vi "CRYO_MASTER_FULL_dev.vi"() -> ()   [LabVIEW 2017]
uses:
  LSI218Data.lvclass
  LSI336Data.lvclass
  USBData.lvclass
  6240AData.lvclass
  DMMsData.lvclass
  LMData.lvclass
  <vilib>/DAQmx/miscellaneous.llb/DAQmx Fill In Error Info.vi
  <vilib>/DAQmx/create/channels.llb/DAQmx Create Channel (DO-Digital Output).vi
  <vilib>/DAQmx/create/channels.llb/DAQmx Create Channel (AO-Voltage-Basic).vi
  <vilib>/express/express arith-compare/Formula/XNode/ExpressFormulaBlockNode.xnode
  <vilib>/Analysis/NI_AALBase.lvlib
  istr.lib/Agilent 33XXX Series/Agilent 33XXX Series.lvlib
panel:
  in  "Automatic \nScreenshots?":bool=TRUE
  in  "Frontpanel screenshots":bool
  in  "Screenshots interval":i64=3605
  in  "Record interval":i64=10
  out "Cycle #":u32
  in  "Measurement Interval (s)":dbl=1.0
  in  "Stop Button":bool
  in  "?":T1(tab)=enum."INST CONFIG"
  out "RUN Identifier":string="20201120_195613_RUNII"
  in  "Base Path (screenshots)":path=path "C:/LabVIEW/DATA/Google/TUCAN Experiments/KEK_cryotests_2019-2020/data/screenshots"
  out "error out (USB6210/6218 AOUT)":errorcluster
  in  "AOUT Labels":string[](array[string])=["PWR400H_I", "PMC183A_I"]
  in  "DOUT Labels":string[](array[string])=["D_V1_NO", "D_V2_NC", "D_CV1", "D_H1"]
  in  "AOUT assignment":tag[](array[tag])=["Dev1/ao0", "Dev1/ao1"]
  out "AO task out":refnum<k21>="20201120_102906_RUNII_AO"
  in  "Analog Out ON?":bool=TRUE
  in  "InstName (USB6218)":string="USB6218"
  in  "USB6218 Config":T2(array[cluster])=[{"Label"="F_1", "FileFormat"="%5.5f", "Active?"=TRUE, "Physical CH"="Dev1/ai0", " terminal\n type"=10083, "ConversionType"={"Type"=enum."SimpleProp", "ConversionParameters"=[0.0, 5.0, 0.0, 500.0]}, "VoltageLimits"=[0.0, 5.0]}, {"Label"="F_2", "FileFormat"="%5.5f", "Active?"=TRUE, "Physical CH"="Dev1/ai1", " terminal\n type"=10083, "ConversionType"={"Type"=enum."SimpleProp", "ConversionParameters"=[0.0, 5.0, 0.0, 200.0]}, "VoltageLimits"=[0.0, 5.0]}, {"Label"="F_3", "FileFormat"="%5.5f", "Active?"=TRUE, "Physical CH"="Dev1/ai2", " terminal\n type"=10083, "ConversionType"={"Type"=enum."SimpleProp", "ConversionParameters"=[0.0, 5.0, 0.0, 200.0]}, "VoltageLimits"=[0.0, 5.0]}, {"Label"="F_4", "FileFormat"="%5.5f", "Active?"=TRUE, "Physical CH"="Dev1/ai3", " terminal\n type"=10083, "ConversionType"={"Type"=enum."SimpleProp", "ConversionParameters"=[0.0, 5.0, 0.0, 500.0]}, "VoltageLimits"=[0.0, 5.0]}, {"Label"="F_5", "FileFormat"="%5.5f", "Active?"=TRUE, "Physical CH"="Dev1/ai4", " terminal\n type"=10083, "ConversionType"={"Type"=enum."SimpleProp", "ConversionParameters"=[0.0, 5.0, 0.0, 500.0]}, "VoltageLimits"=[0.0, 5.0]}, {"Label"="I_CV", "FileFormat"="%3.5f", "Active?"=TRUE, "Physical CH"="Dev1/ai5", " terminal\n type"=10083, "ConversionType"={"Type"=enum."Raw", "ConversionParameters"=[0.0, 0.0, 0.0, 0.0]}, "VoltageLimits"=[0.0, 10.0]}, {"Label"="CV1_answer", "FileFormat"="%3.5f", "Active?"=TRUE, "Physical CH"="Dev1/ai6", " terminal\n type"=10083, "ConversionType"={"Type"=enum."SimpleProp", "ConversionParameters"=[1.0, 5.0, 0.0, 100.0]}, "VoltageLimits"=[0.0, 5.0]}, {"Label"="P_Dewar", "FileFormat"="%5.5e", "Active?"=TRUE, "Physical CH"="Dev1/ai7", " terminal\n type"=10083, "ConversionType"={"Type"=enum."SimpleProp", "ConversionParameters"=[1.0, 5.0, 0.0, 200000.0]}, "VoltageLimits"=[0.0, 5.0]}] {"terminal\n type" items=["Default"=-1, "RSE"=10083, "NRSE"=10078, "Differential"=10106, "Pseudodifferential"=12529]}
  out "error out (USB6218)":errorcluster
  out "error out (USB6210/6218 DOUT)":errorcluster={"status"=TRUE, "code"=-200428, "source"="CRYO_MASTER_FULL_dev.vi<append>\n<B>Task Name: </B>20201120_102906_DO"}
  out "DOUT task out":refnum<k21>="20201120_102906_DO"
  in  "DOUT Physical CH":tag[](array[tag])=["Dev1/port1/line0", "Dev1/port1/line1", "Dev1/port1/line2", "Dev1/port1/line3"]
  in  "Digital Out ON?":bool=TRUE
  in  "USB6210 Config":T2(array[cluster])=[{"Label"="P_ins", "FileFormat"="%5.5e", "Active?"=TRUE, "Physical CH"="Dev2/ai0", " terminal\n type"=10083, "ConversionType"={"Type"=enum."CC-10_LOG", "ConversionParameters"=[0.5, 9.0, 0.0, 1.0]}, "VoltageLimits"=[0.0, 10.0]}, {"Label"="P_4Kres", "FileFormat"="%5.5e", "Active?"=TRUE, "Physical CH"="Dev2/ai1", " terminal\n type"=10083, "ConversionType"={"Type"=enum."SimpleProp", "ConversionParameters"=[1.0, 5.0, 0.0, 200000.0]}, "VoltageLimits"=[0.0, 5.0]}, {"Label"="P_3HeIN", "FileFormat"="%5.5e", "Active?"=TRUE, "Physical CH"="Dev2/ai2", " terminal\n type"=10083, "ConversionType"={"Type"=enum."SimpleProp", "ConversionParameters"=[1.0, 5.0, 0.0, 200000.0]}, "VoltageLimits"=[0.0, 5.0]}, {"Label"="P_SldRTN", "FileFormat"="%5.5e", "Active?"=TRUE, "Physical CH"="Dev2/ai3", " terminal\n type"=10083, "ConversionType"={"Type"=enum."SimpleProp", "ConversionParameters"=[1.0, 5.0, 0.0, 200000.0]}, "VoltageLimits"=[0.0, 5.0]}, {"Label"="P_3Hepot", "FileFormat"="%5.5e", "Active?"=TRUE, "Physical CH"="Dev2/ai4", " terminal\n type"=10083, "ConversionType"={"Type"=enum."SimpleProp", "ConversionParameters"=[0.0, 10.0, 0.0, 133320.0]}, "VoltageLimits"=[0.0, 10.0]}, {"Label"="P_1Kpot", "FileFormat"="%5.5e", "Active?"=TRUE, "Physical CH"="Dev2/ai5", " terminal\n type"=10083, "ConversionType"={"Type"=enum."SimpleProp", "ConversionParameters"=[0.0, 10.0, 0.0, 133320.0]}, "VoltageLimits"=[0.0, 10.0]}, {"Label"="P_Dewar(old)", "FileFormat"="%5.5e", "Active?"=FALSE, "Physical CH"="Dev2/ai6", " terminal\n type"=10083, "ConversionType"={"Type"=enum."SimpleProp", "ConversionParameters"=[1.0, 5.0, 0.0, 200000.0]}, "VoltageLimits"=[0.0, 5.0]}, {"Label"="DP_HEX4", "FileFormat"="%5.5e", "Active?"=TRUE, "Physical CH"="Dev2/ai7", " terminal\n type"=10083, "ConversionType"={"Type"=enum."SimpleProp", "ConversionParameters"=[1.0, 5.0, 0.0, 1000.0]}, "VoltageLimits"=[0.0, 5.0]}, {"Label"="DP_HEX5", "FileFormat"="%5.5e", "Active?"=TRUE, "Physical CH"="Dev2/ai8", " terminal\n type"=10083, "ConversionType"={"Type"=enum."SimpleProp", "ConversionParameters"=[1.0, 5.0, 0.0, 1000.0]}, "VoltageLimits"=[0.0, 5.0]}, {"Label"="L1(old)", "FileFormat"="%5.5f", "Active?"=TRUE, "Physical CH"="Dev2/ai9", " terminal\n type"=10083, "ConversionType"={"Type"=enum."SimpleProp", "ConversionParameters"=[0.0, 10.0, 0.0, 100.0]}, "VoltageLimits"=[0.0, 10.0]}, {"Label"="L2-1", "FileFormat"="%5.5f", "Active?"=TRUE, "Physical CH"="Dev2/ai10", " terminal\n type"=10083, "ConversionType"={"Type"=enum."SimpleProp", "ConversionParameters"=[0.0, 10.0, 0.0, 100.0]}, "VoltageLimits"=[0.0, 10.0]}, {"Label"="L2-2", "FileFormat"="%5.5f", "Active?"=TRUE, "Physical CH"="Dev2/ai11", " terminal\n type"=10083, "ConversionType"={"Type"=enum."SimpleProp", "ConversionParameters"=[0.0, 10.0, 0.0, 100.0]}, "VoltageLimits"=[0.0, 10.0]}, {"Label"="L3", "FileFormat"="%5.5f", "Active?"=TRUE, "Physical CH"="Dev2/ai12", " terminal\n type"=10083, "ConversionType"={"Type"=enum."SimpleProp", "ConversionParameters"=[0.0, 10.0, 0.0, 100.0]}, "VoltageLimits"=[0.0, 10.0]}, {"Label"="P_HEX7OUT", "FileFormat"="%5.5e", "Active?"=TRUE, "Physical CH"="Dev2/ai13", " terminal\n type"=10083, "ConversionType"={"Type"=enum."SimpleProp", "ConversionParameters"=[1.0, 5.0, 0.0, 200000.0]}, "VoltageLimits"=[0.0, 5.0]}, {"Label"="P_IP", "FileFormat"="%5.5e", "Active?"=TRUE, "Physical CH"="Dev2/ai14", " terminal\n type"=10083, "ConversionType"={"Type"=enum."CC-10_LOG", "ConversionParameters"=[0.5, 9.0, 0.0, 1.0]}, "VoltageLimits"=[0.0, 10.0]}, {"Label"="V_H1", "FileFormat"="%3.5f", "Active?"=TRUE, "Physical CH"="Dev2/ai15", " terminal\n type"=10083, "ConversionType"={"Type"=enum."Raw", "ConversionParameters"=[0.0, 1.0, 0.0, 1.0]}, "VoltageLimits"=[0.0, 10.0]}] {"terminal\n type" items=["Default"=-1, "RSE"=10083, "NRSE"=10078, "Differential"=10106, "Pseudodifferential"=12529]}
  in  "RUN label":string="RUNII"
  in  "Base Path":path=path "C:/LabVIEW/DATA/RUN_2"
  in  "InstName (USB6210)":string="USB6210"
  out "error out (USB6210)":errorcluster
  out "File Refn USB AO":refnum<file>
  out "File Refn USB DO":refnum<file>
  in  "LM measurement interval (>0)":i64=1
  in  "Active? (HP34401 LM)":bool=TRUE
  in  "Labels (HP34401 LM)":string[](array[string])=["R_L1", "L1"]
  in  "FileFormat (HP34401 LM)":string[](array[string])=["%.4f", "%.4f"]
  in  "VISA (HP34401 LM)":refnum<visa-resource-name>="GPIB0::24::INSTR"
  in  "LevelCalibration (R0, R1, L0, L1)":dbl[](array[numeric])=[179.74, 0.0, 0.0, 100.0]
  in  "InstName (HP34401 LM)":string="HP34401LM"
  out "error out (LSI336)":errorcluster
  in  "InstName (LSI336)":string="LSI336"
  in  "FileFormat (336)":string="%4.4f"
  in  "LSI336Settings(X,Y)":T3(array[cluster])=[{"LSIName"="LSi336X", "Labels"=["T1K3-1", "T1K3-2", "T3He5", "T3He8"], "SensorLocations"=[enum."T1K3-1", enum."T1K3-2", enum."T3He5", enum."T3He8"], "Active?"=TRUE, "VISA res. name"="COM15_LSI336Y"}, {"LSIName"="LSi336Y", "Labels"=["T3He6-1", "T3He6-2", "T3He7-1", "T3He7-2"], "SensorLocations"=[enum."T3He6-1", enum."T3He6-2", enum."T3He7-1", enum."T3He7-2"], "Active?"=TRUE, "VISA res. name"="COM20_LSI336X"}]
  in  "FileFormat (218)":string="%4.4f"
  in  "InstName (LSI218)":string="LSI218"
  in  "LSI218Settings(A-F)":T3(array[cluster])=[{"LSIName"="LSI218A", "Labels"=["T3He10", "T3He1-1", "TTH3", "TTH4", "TTH1", "TTH2", "T4He1", "T1K1"], "SensorLocations"=[enum."T3He10", enum."T3He1-1", enum."TTH3", enum."TTH4", enum."TTH1", enum."TTH2", enum."T4He1", enum."T1K1"], "Active?"=TRUE, "VISA res. name"="GPIB0::7::INSTR"}, {"LSIName"="LSI218B", "Labels"=["N.C.", "N.C.", "N.C.", "N.C.", "T3He2-1", "T3He2-2", "T3He3", "T3He1-4"], "SensorLocations"=[enum."N.C.", enum."N.C.", enum."N.C.", enum."N.C.", enum."T3He2-1", enum."T3He2-2", enum."T3He3", enum."T3He1-4"], "Active?"=TRUE, "VISA res. name"="GPIB0::4::INSTR"}, {"LSIName"="LSI218C", "Labels"=["T4He3-1", "T4He3-2", "T4He3-3", "T4He3-4", "T4He2-1", "T4He2-2", "T4He4", "T4He5"], "SensorLocations"=[enum."T4He3-1", enum."T4He3-2", enum."T4He3-3", enum."T4He3-4", enum."T4He2-1", enum."T4He2-2", enum."T4He4", enum."T4He5"], "Active?"=TRUE, "VISA res. name"="GPIB0::3::INSTR"}, {"LSIName"="LSI218D", "Labels"=["T4He6", "T4He9", "T3He1-2", "T3He1-3", "T4He7", "T4He8", "T4He10", "T1K6"], "SensorLocations"=[enum."T4He6", enum."T4He9", enum."T3He1-2", enum."T3He1-3", enum."T4He7", enum."T4He8", enum."T4He10", enum."T1K6"], "Active?"=TRUE, "VISA res. name"="GPIB0::5::INSTR"}, {"LSIName"="LSI218E", "Labels"=["TIP1", "N.C.", "TIP2", "N.C.", "TIP3", "TIP4", "TIP5", "N.C."], "SensorLocations"=[enum."TIP1", enum."N.C.", enum."TIP2", enum."N.C.", enum."TIP3", enum."TIP4", enum."TIP5", enum."N.C."], "Active?"=TRUE, "VISA res. name"="GPIB0::11::INSTR"}, {"LSIName"="LSI218F", "Labels"=["T1K2", "T1K4", "T1K5", "T3He4", "T3He9", "TIP6", "N.C.", "N.C."], "SensorLocations"=[enum."T1K2", enum."T1K4", enum."T1K5", enum."T3He4", enum."T3He9", enum."TIP6", enum."N.C.", enum."N.C."], "Active?"=TRUE, "VISA res. name"="GPIB0::8::INSTR"}]
  out "error out (LSI218)":errorcluster
  out "RUN Identifier 2":string="20201120_195613_RUNII" caption="RUN Identifier"
  out "error out (HP34401 LM)":errorcluster
  out "Graph 3":T4(graph) caption="XY Graph"
  out "Graph 1":T4(graph) caption="XY Graph"
  in  "FIle suffix 4":string="Graph4_noise"
  in  "Take Screenshot! 4":bool
  in  "Take Screenshot! 3":bool
  in  "Take Screenshot! 2":bool
  in  "Take Screenshot! 1":bool
  in  "FIle suffix 3":string="Graph3_noise"
  in  "FIle suffix 2":string="Graph2_noise"
  in  "FIle suffix 1":string="Graph1_noise"
  in  "log/linear 2":bool
  in  "Tab Control 2":T5(tab)
  in  "Plot selecter (USB6210)\n    1      2     3     4":bool[][](array[boolean])=[[TRUE, FALSE, FALSE, FALSE], [TRUE, FALSE, FALSE, FALSE], [TRUE, FALSE, FALSE, FALSE], [TRUE, FALSE, FALSE, FALSE], [TRUE, FALSE, FALSE, FALSE], [TRUE, FALSE, FALSE, FALSE], [TRUE, FALSE, FALSE, FALSE], [FALSE, TRUE, FALSE, FALSE], [FALSE, TRUE, FALSE, FALSE], [FALSE, TRUE, FALSE, FALSE], [FALSE, TRUE, FALSE, FALSE], [FALSE, TRUE, FALSE, FALSE], [FALSE, TRUE, FALSE, FALSE], [TRUE, FALSE, FALSE, FALSE], [TRUE, FALSE, FALSE, FALSE], [FALSE, FALSE, FALSE, FALSE]]
  out "All Labels (USB6210)":string[](array[string])=["P_ins", "P_4Kres", "P_3HeIN", "P_SldRTN", "P_3Hepot", "P_1Kpot", "P_Dewar(old)", "DP_HEX4", "DP_HEX5", "L1", "L2-1", "L2-2", "L3", "P_HEX7OUT", "P_IP", "V_H1"]
  out "Last Data \n(USB6210)":dbl[](array[numeric])=[0.00014344236967610548, 99965.74495067913, 99950.94515133197, 99352.37411946112, 99886.7829519446, 100189.26718267406, 0.0, -43.427572689286905, 129.38299172882833, 0.2500313879300094, 49.82195192384119, 46.222738577499655, -0.009730557048235056, 99939.4341328877, 0.0001425329978286714, 5.7259116978123625] format="%#_6e"
  out "Time of Last Measurement (USB6210)":timestamp=timestamp(3688714213.5022345 s since 1904-01-01)
  out "USB6210 Status":T6(ring)=enum."Ready"
  out "Last Vol\n(USB6210)":dbl[](array[numeric])=[5.578338725591466, 2.9993148990135827, 2.999018903026639, 2.9870474823892224, 7.492257947190564, 7.51494653335389, 0.0, 0.8262897092428524, 1.5175319669153133, 0.02500313879300094, 4.982195192384119, 4.622273857749965, -0.0009730557048235056, 2.998788682657754, 5.576957709771981, 5.7259116978123625] format="%_5f"
  out "Labels (HP34401 LM) 2":string[](array[string])=["R_L1", "L1"]
  out "LastData (HP34401 LM)":dbl[](array[numeric])
  in  "Plot selecter (HP34401A)\n    1      2     3     4":bool[][](array[boolean])=[[TRUE, FALSE, FALSE, FALSE], [TRUE, FALSE, FALSE, FALSE], [TRUE, FALSE, FALSE, FALSE], [TRUE, FALSE, FALSE, FALSE], [TRUE, FALSE, FALSE, FALSE], [TRUE, FALSE, FALSE, FALSE], [TRUE, FALSE, FALSE, FALSE], [FALSE, TRUE, FALSE, FALSE], [FALSE, TRUE, FALSE, FALSE], [FALSE, TRUE, FALSE, FALSE], [FALSE, TRUE, FALSE, FALSE], [FALSE, TRUE, FALSE, FALSE], [FALSE, TRUE, FALSE, FALSE], [TRUE, FALSE, FALSE, FALSE], [TRUE, FALSE, FALSE, FALSE], [FALSE, FALSE, FALSE, FALSE]]
  out "Time of Last Measurement (USB6218)":timestamp=timestamp(3688714213.512236 s since 1904-01-01)
  out "USB6218 Status":T6(ring)=enum."Ready"
  out "Last Vol \n(USB6218)":dbl[](array[numeric])=[0.027353351515475806, -0.0023691627670037628, 0.005620406973829139, -0.06395132134572999, 0.37813814934166257, 0.26085215700955067, -0.0017444638941784426, 3.020512761209526] format="%_5f"
  out "Last Data \n(USB6218)":dbl[](array[numeric])=[2.735335151547581, -0.09476651068015052, 0.22481627895316558, -6.395132134572999, 37.81381493416626, 0.26085215700955067, -25.04361159735446, 101025.63806047631] format="%#_6e"
  out "All Labels (USB6218)":string[](array[string])=["F_1", "F_2", "F_3", "F_4", "F_5", "I_CV", "CV1_answer", "P_Dewar"]
  in  "Plot selecter (USB6218)\n    1      2     3     4":bool[][](array[boolean])=[[FALSE, FALSE, TRUE, FALSE], [FALSE, FALSE, TRUE, FALSE], [FALSE, FALSE, TRUE, FALSE], [FALSE, FALSE, TRUE, FALSE], [FALSE, FALSE, TRUE, FALSE], [FALSE, FALSE, TRUE, FALSE], [FALSE, FALSE, FALSE, FALSE], [FALSE, FALSE, TRUE, FALSE], [FALSE, FALSE, TRUE, FALSE], [FALSE, FALSE, FALSE, TRUE], [FALSE, FALSE, FALSE, TRUE], [FALSE, FALSE, FALSE, TRUE], [FALSE, FALSE, FALSE, TRUE], [FALSE, FALSE, FALSE, FALSE], [FALSE, FALSE, FALSE, FALSE], [FALSE, FALSE, FALSE, FALSE]]
  out "Time of Last Measurement (LSI218)":timestamp=timestamp(3688714213.494224 s since 1904-01-01)
  out "LSI218 Status":T7(ring)=enum."Measuring"
  out "Last Data \nLSI218 (1)":dbl[](array[numeric])=[250.64, 279.64, 106.3, 112.52, 19.165, 19.038, 4.436, 10.775, 30.0, 0.0, 0.0, 0.0, 46.025, 34.792, 17.25, 276.96, 287.74, 287.84, 285.5, 285.55, 34.292, 35.074, 30.928, 25.728]
  out "Labels LSI218 (1)":string[](array[string])=["T3He10", "T3He1-1", "TTH3", "TTH4", "TTH1", "TTH2", "T4He1", "T1K1", "N.C.", "N.C.", "N.C.", "N.C.", "T3He2-1", "T3He2-2", "T3He3", "T3He1-4", "T4He3-1", "T4He3-2", "T4He3-3", "T4He3-4", "T4He2-1", "T4He2-2", "T4He4", "T4He5"]
  in  "Plot selecter LSI218(1)\n    1      2     3     4":bool[][](array[boolean])=[[FALSE, FALSE, FALSE, FALSE], [FALSE, FALSE, FALSE, FALSE], [FALSE, FALSE, FALSE, TRUE], [FALSE, FALSE, FALSE, TRUE], [FALSE, FALSE, FALSE, TRUE], [FALSE, FALSE, FALSE, TRUE], [FALSE, FALSE, FALSE, TRUE], [FALSE, FALSE, FALSE, TRUE], [FALSE, FALSE, FALSE, FALSE], [FALSE, FALSE, FALSE, FALSE], [FALSE, FALSE, FALSE, FALSE], [FALSE, FALSE, FALSE, FALSE], [FALSE, FALSE, FALSE, TRUE], [FALSE, FALSE, FALSE, TRUE], [FALSE, FALSE, FALSE, FALSE], [FALSE, FALSE, FALSE, FALSE], [FALSE, FALSE, FALSE, TRUE], [FALSE, FALSE, FALSE, TRUE], [FALSE, FALSE, FALSE, TRUE], [FALSE, FALSE, FALSE, TRUE], [FALSE, FALSE, FALSE, TRUE], [FALSE, FALSE, FALSE, TRUE], [FALSE, FALSE, FALSE, TRUE], [FALSE, FALSE, FALSE, FALSE]]
  out "Active?\n (1)":bool[](array[boolean])=[TRUE, TRUE, TRUE, TRUE, TRUE, TRUE, TRUE, TRUE, TRUE, TRUE, TRUE, TRUE, TRUE, TRUE, TRUE, TRUE, TRUE, TRUE, TRUE, TRUE, TRUE, TRUE, TRUE, TRUE]
  out "Labels LSI218 (2)":string[](array[string])=["T4He6", "T4He9", "T3He1-2", "T3He1-3", "T4He7", "T4He8", "T4He10", "T1K6", "TIP1", "N.C.", "TIP2", "N.C.", "TIP3", "TIP4", "TIP5", "N.C.", "T1K2", "T1K4", "T1K5", "T3He4", "T3He9", "TIP6", "N.C.", "N.C."]
  out "Active?\n(2)":bool[](array[boolean])=[TRUE, TRUE, TRUE, TRUE, TRUE, TRUE, TRUE, TRUE, TRUE, TRUE, TRUE, TRUE, TRUE, TRUE, TRUE, TRUE, TRUE, TRUE, TRUE, TRUE, TRUE, TRUE, TRUE, TRUE]
  out "Last Data \nLSI218 (2)":dbl[](array[numeric])=[25.125, 97.886, 279.52, 277.53, 115.69, 166.07, 208.39, 250.44, 246.21, 0.0, 88.2, 688.49, 39.062, 11.046, 17.368, 688.58, 4.194, 4.476, 4.691, 9.636, 10.639, 18.262, 0.433, 0.0]
  in  "Plot selecter LSI218(2)\n    1      2     3     4":bool[][](array[boolean])=[[FALSE, FALSE, FALSE, FALSE], [FALSE, FALSE, FALSE, FALSE], [FALSE, FALSE, FALSE, FALSE], [FALSE, FALSE, FALSE, FALSE], [FALSE, FALSE, FALSE, FALSE], [FALSE, FALSE, FALSE, FALSE], [FALSE, FALSE, FALSE, FALSE], [FALSE, FALSE, FALSE, FALSE], [FALSE, FALSE, FALSE, FALSE], [FALSE, FALSE, FALSE, FALSE], [FALSE, FALSE, FALSE, FALSE], [FALSE, FALSE, FALSE, FALSE], [FALSE, FALSE, FALSE, FALSE], [FALSE, FALSE, FALSE, FALSE], [FALSE, FALSE, FALSE, FALSE], [FALSE, FALSE, FALSE, FALSE], [FALSE, FALSE, FALSE, TRUE], [FALSE, FALSE, FALSE, TRUE], [FALSE, FALSE, FALSE, TRUE], [FALSE, FALSE, FALSE, TRUE], [FALSE, FALSE, FALSE, FALSE], [FALSE, FALSE, FALSE, FALSE], [FALSE, FALSE, FALSE, FALSE], [FALSE, FALSE, FALSE, FALSE]]
  in  "Plot selecter LSI336 \n     1      2     3     4":bool[][](array[boolean])=[[FALSE, FALSE, FALSE, TRUE], [FALSE, FALSE, FALSE, TRUE], [FALSE, FALSE, FALSE, TRUE], [FALSE, FALSE, FALSE, TRUE], [FALSE, FALSE, FALSE, TRUE], [FALSE, FALSE, FALSE, TRUE], [FALSE, FALSE, FALSE, TRUE], [FALSE, FALSE, FALSE, TRUE]]
  out "Time of Last Measurement (LSI336)":timestamp=timestamp(3688714213.494224 s since 1904-01-01)
  out "Last Data \nLSI336":dbl[](array[numeric])=[4.182, 4.1886, 4.3213, 8.8312, 8.4926, 8.5004, 8.4614, 8.3712]
  out "Active?\n(LSI336)":bool[](array[boolean])=[TRUE, TRUE, TRUE, TRUE, TRUE, TRUE, TRUE, TRUE]
  out "Labels LSI336":string[](array[string])=["T1K3-1", "T1K3-2", "T3He5", "T3He8", "T3He6-1", "T3He6-2", "T3He7-1", "T3He7-2"]
  out "LSI336 Status":T7(ring)=enum."Measuring"
  in  "log/linear 1":bool
  out "Graph 2":T4(graph) caption="XY Graph"
  out "Graph 4":T4(graph) caption="XY Graph"
  in  "log/linear 4":bool
  in  "log/linear 3":bool
  out "RUN Identifier 3":string="20201120_195613_RUNII" caption="RUN Identifier"
  in  "AutoFill Source (P)":T8(ring)=enum."USB6218AI"
  in  "AutoFill Source (L)":T8(ring)
  out "RUN Identifier 4":string="20201120_195613_RUNII" caption="RUN Identifier"
  out "Fill (false)":bool=TRUE
  in  "Fill state":bool
  out "state 1 (false)":bool
  out "state 1":bool=TRUE
  out "state 2":bool=TRUE
  out "state 2 (false)":bool
  out "Status V2 CTRL":enum16{"Pressurize", "Release"}(ring)=enum."Release"
  out "Status V1 CTRL":enum16{"Pressurize", "Release"}(ring)
  out "Lav (%)":dbl=68.6437257114393 format="%0.2f"
  out "Lstd":dbl=0.0368003341020671 format="%0.2f"
  out "Last N M.A. Levels":dbl[](array[numeric])=[68.66350181207783, 68.66925614084933, 68.66350181209265, 68.65824071145909, 68.66432385894117, 68.66498149652449, 68.66333740270238, 68.6659679529995, 68.65873393973654, 68.66021362426311, 68.63949804138589, 68.6057941170069, 68.58474971550248, 68.55005933460893] format="%_5e"
  out "Lstd history":dbl(graph)=0.025405513884442257
  out "Lav history":dbl(graph)=68.65206361610068
  out "Target Index (L)":i32=12
  in  "Auto Fll He L. label":string="L3"
  out "Target Index (P)":i32=7
  in  "Auto Fll Dewar P. label":string="P_Dewar"
  out "He Level":T9(graph)=[{"TimeArray"=[timestamp(3688681440.5182567 s since 1904-01-01), timestamp(3688681441.528362 s since 1904-01-01), timestamp(3688681442.529063 s since 1904-01-01), timestamp(3688681443.5308065 s since 1904-01-01), timestamp(3688681444.533836 s since 1904-01-01), timestamp(3688681445.5861793 s since 1904-01-01), timestamp(3688681446.586079 s since 1904-01-01), timestamp(3688681447.585863 s since 1904-01-01), timestamp(3688681448.5861926 s since 1904-01-01), timestamp(3688681449.585548 s since 1904-01-01), timestamp(3688681451.1870184 s since 1904-01-01), timestamp(3688681452.1881447 s since 1904-01-01), timestamp(3688681453.1869626 s since 1904-01-01), timestamp(3688681454.1869583 s since 1904-01-01)], "Filtered X"=[68.64475914147651, 68.67501046951253, 68.65330842954738, 68.65988480529988, 68.6690917314049, 68.67764101984578, 68.64673205425893, 68.67040700648839, 68.64015567835303, 68.68355975795208, 68.56386972275008, 68.53559130897234, 68.55597807233536, 68.54479823437791]}, {"TimeArray"=[timestamp(3688681440.5182567 s since 1904-01-01), timestamp(3688681441.528362 s since 1904-01-01), timestamp(3688681442.529063 s since 1904-01-01), timestamp(3688681443.5308065 s since 1904-01-01), timestamp(3688681444.533836 s since 1904-01-01), timestamp(3688681445.5861793 s since 1904-01-01), timestamp(3688681446.586079 s since 1904-01-01), timestamp(3688681447.585863 s since 1904-01-01), timestamp(3688681448.5861926 s since 1904-01-01), timestamp(3688681449.585548 s since 1904-01-01), timestamp(3688681451.1870184 s since 1904-01-01), timestamp(3688681452.1881447 s since 1904-01-01), timestamp(3688681453.1869626 s since 1904-01-01), timestamp(3688681454.1869583 s since 1904-01-01)], "Filtered X"=[68.66350181207783, 68.66925614084933, 68.66350181209265, 68.65824071145909, 68.66432385894117, 68.66498149652449, 68.66333740270238, 68.6659679529995, 68.65873393973654, 68.66021362426311, 68.63949804138589, 68.6057941170069, 68.58474971550248, 68.55005933460893]}] caption="XY Graph"
  in  "P_safelimit_high (Pa)":dbl=300000.0 format="%_4e"
  in  "P_safelimit_low (Pa)":dbl=100.0 format="%_4e"
  in  "Auto Fill ON?":bool
  out "Pstd history":dbl(graph)=114.38812118954785
  out "Pav history":dbl(graph)=105675.35030459762
  in  "Mov. Avg Interval":i64=4
  in  "V2 (N.C.)":bool
  in  "V1 (N.O.)":bool=TRUE
  in  "N for sampling":i64=7
  in  "L_low (%)":dbl=60.0 format="%_3f"
  in  "L_high (%)":dbl=80.0 format="%_3g"
  in  "P_2_low (Pa)":dbl=115000.0 format="%_4e"
  in  "P_1_low (Pa)":dbl=120000.0 format="%_4g"
  in  "P_2_high (Pa)":dbl=120000.0 format="%_4e"
  in  "P_1_high (Pa)":dbl=132000.0 format="%_4e"
  out "Dewar Pressure":T9(graph)=[{"TimeArray"=[timestamp(3688681440.5182567 s since 1904-01-01), timestamp(3688681441.528362 s since 1904-01-01), timestamp(3688681442.529063 s since 1904-01-01), timestamp(3688681443.5308065 s since 1904-01-01), timestamp(3688681444.533836 s since 1904-01-01), timestamp(3688681445.5861793 s since 1904-01-01), timestamp(3688681446.586079 s since 1904-01-01), timestamp(3688681447.585863 s since 1904-01-01), timestamp(3688681448.5861926 s since 1904-01-01), timestamp(3688681449.585548 s since 1904-01-01), timestamp(3688681451.1870184 s since 1904-01-01), timestamp(3688681452.1881447 s since 1904-01-01), timestamp(3688681453.1869626 s since 1904-01-01), timestamp(3688681454.1869583 s since 1904-01-01)], "Filtered X"=[105179.8781041116, 106057.74282245144, 105580.99980780583, 106041.30340772575, 105400.16625394224, 105776.62883990775, 106128.43230131528, 105580.99980910066, 105599.08316388502, 105337.69648153422, 106230.35666842951, 105848.96226133379, 105405.09807586943, 105922.93962293878]}, {"TimeArray"=[timestamp(3688681440.5182567 s since 1904-01-01), timestamp(3688681441.528362 s since 1904-01-01), timestamp(3688681442.529063 s since 1904-01-01), timestamp(3688681443.5308065 s since 1904-01-01), timestamp(3688681444.533836 s since 1904-01-01), timestamp(3688681445.5861793 s since 1904-01-01), timestamp(3688681446.586079 s since 1904-01-01), timestamp(3688681447.585863 s since 1904-01-01), timestamp(3688681448.5861926 s since 1904-01-01), timestamp(3688681449.585548 s since 1904-01-01), timestamp(3688681451.1870184 s since 1904-01-01), timestamp(3688681452.1881447 s since 1904-01-01), timestamp(3688681453.1869626 s since 1904-01-01), timestamp(3688681454.1869583 s since 1904-01-01)], "Filtered X"=[105428.11325729526, 105625.3862278013, 105622.09834564029, 105714.98103552366, 105770.05307298132, 105699.7745773454, 105836.63270072275, 105721.55680106647, 105771.28602855216, 105661.55293895879, 105687.03403073736, 105754.02464379564, 105705.52837179173, 105851.83915714288]}] caption="XY Graph"
  out "Last N M.A. Pressures":dbl[](array[numeric])=[105428.11325729526, 105625.3862278013, 105622.09834564029, 105714.98103552366, 105770.05307298132, 105699.7745773454, 105836.63270072275, 105721.55680106647, 105771.28602855216, 105661.55293895879, 105687.03403073736, 105754.02464379564, 105705.52837179173, 105851.83915714288] format="%_5e"
  out "Pav (Pa)":dbl=105703.56151352536 format="%0.4e"
  out "Pstd":dbl=104.65259509003522 format="%0.4e"
  out "File Refn DewarCTRL":refnum<file>
  out "Error Out (Dewar CTRL":errorcluster
  in  "lower limit (mA) \n(PMC)":dbl=4.0 format="%_3f"
  in  "upper limit (mA)\n (PMC)":dbl=40.0 format="%_3f"
  in  "OUTPUT\n(PMC)":bool
  in  "Set Current (mA)\n (PMC)":dbl=4.0 min=4.0 max=40.0 format="%_3g"
  in  "update values":bool
  out "Monitor Current (mA)":dbl=3.4351617247063078 min=0.0 max=1.9 format="%_4e"
  in  "update current":bool
  out "USB 6218 AOUT":dbl[](array[numeric])=[0.004, 0.004, 0.06969546425555169, 0.06969546425555169]
  out "Graph 7":T10(graph) caption="XY Graph"
  in  "lower limit (mA) \n(PWR)":dbl=4.0 format="%_3f"
  in  "upper limit (mA)\n (PWR)":dbl=20.0 format="%_3f"
  in  "lower limit (mA)":dbl=4.0 format="%_3f"
  in  "SetCurrent 2 (mA)":dbl=4.0 min=4.0 max=500.0 format="%_3f"
  in  "upper limit (mA)":dbl=500.0 format="%_3f"
  out "error out (KIKUSI CTRL)":errorcluster
  out "ActualVoltage (V)":dbl[](array[numeric]) format="%_6g"
  out "ActualCurrent (A)":dbl[](array[numeric]) format="%_3e"
  in  "SetCurrent 1 (mA)":dbl=4.0 min=4.0 max=500.0 format="%_3g"
  in  "Output\n (ADCMT)":bool[](array[boolean])=[FALSE, FALSE]
  out "error out (ADCMT6420A)":errorcluster={"status"=TRUE, "code"=-1073807265, "source"="VISA Write in ADCMT 6240.lvlib:Configure Output Mode (DC).vi->6240AData.lvclass:6240AData_execute.vi->CRYO_MASTER_FULL_dev.vi"}
  in  "Voltage limits (V)":dbl[](array[numeric])=[12.0, 12.0] format="%_3f"
  in  "CtrlLabels":string[](array[string])=["CV2", "CV3"]
  in  "VISA":refnum<visa-resource-name>[](array[refnum])=["GPIB0::1::INSTR", "GPIB0::12::INSTR"]
  out "Initialized?":bool=TRUE
  in  "InstName":string="ADCMT6240"
  out "Graph 6":T9(graph)=[{"TimeArray"=[timestamp(3688680600.1117425 s since 1904-01-01), timestamp(3688680604.613425 s since 1904-01-01), timestamp(3688688430.813075 s since 1904-01-01), timestamp(3688691144.2088265 s since 1904-01-01), timestamp(3688698668.129616 s since 1904-01-01)], "Filtered X"=[0.004, 0.004, 0.018, 0.004, 0.004]}, {"TimeArray"=[timestamp(3688680600.1117425 s since 1904-01-01), timestamp(3688680604.613425 s since 1904-01-01), timestamp(3688688430.813075 s since 1904-01-01), timestamp(3688691144.2088265 s since 1904-01-01), timestamp(3688698668.129616 s since 1904-01-01)], "Filtered X"=[0.02, 0.02, 0.02, 0.02, 0.004]}, {"TimeArray"=[timestamp(3688680600.1117425 s since 1904-01-01), timestamp(3688680604.613425 s since 1904-01-01), timestamp(3688688430.813075 s since 1904-01-01), timestamp(3688691144.2088265 s since 1904-01-01), timestamp(3688698668.129616 s since 1904-01-01)], "Filtered X"=[0.004, 0.004, 0.018, 0.004, 0.004]}, {"TimeArray"=[timestamp(3688680600.1117425 s since 1904-01-01), timestamp(3688680604.613425 s since 1904-01-01), timestamp(3688688430.813075 s since 1904-01-01), timestamp(3688691144.2088265 s since 1904-01-01), timestamp(3688698668.129616 s since 1904-01-01)], "Filtered X"=[0.02, 0.02, 0.02, 0.02, 0.004]}] caption="XY Graph"
  in  "Initialize":bool
  in  "CONTROL KIKUSUI?":bool=TRUE
  in  "OUTPUT\n(PWR)":bool
  in  "Set Current (mA)\n (PWR)":dbl=4.0 min=4.0 max=20.0 format="%_3g"
  out "RUN Identifier 5":string="20201120_195613_RUNII" caption="RUN Identifier"
  out "ƒ¢T=T_2 -T_1":dbl
  out "Graph DMMs 3":T4(graph) caption="XY Graph"
  out "Q = I *V":dbl
  in  "index I":i64
  in  "index V":i64=1
  out "VariableSources":T11(array[ring])
  in  "DMMsConfig (variables)":T12(array[cluster])=[{"Label"="P_3Hepot", "Active?"=TRUE, "Source"=enum."USB6210", "SourceLabel"="P_3Hepot", "FileFormat"="%6.4e"}, {"Label"="F_1", "Active?"=TRUE, "Source"=enum."USB6218AI", "SourceLabel"="F_1", "FileFormat"="%3.4f"}, {"Label"="F_4", "Active?"=TRUE, "Source"=enum."USB6218AI", "SourceLabel"="F_4", "FileFormat"="%3.4f"}, {"Label"="F_5", "Active?"=TRUE, "Source"=enum."USB6218AI", "SourceLabel"="F_5", "FileFormat"="%3.4f"}, {"Label"="DP_HEX4", "Active?"=TRUE, "Source"=enum."USB6210", "SourceLabel"="DP_HEX4", "FileFormat"="%4.3e"}, {"Label"="T3He6-1", "Active?"=TRUE, "Source"=enum."LSI336", "SourceLabel"="T3He6-1", "FileFormat"="%3.4f"}, {"Label"="T3He6-2", "Active?"=TRUE, "Source"=enum."LSI336", "SourceLabel"="T3He6-2", "FileFormat"="%3.4f"}, {"Label"="T3He7-1", "Active?"=TRUE, "Source"=enum."LSI336", "SourceLabel"="T3He7-1", "FileFormat"="%3.4f"}, {"Label"="T3He7-2", "Active?"=TRUE, "Source"=enum."LSI336", "SourceLabel"="T3He7-2", "FileFormat"="%3.4f"}]
  in  "Measure DMMs?":bool=TRUE
  out "DMMsLabels":string[](array[string])
  out "Active?":bool[](array[boolean])
  out "DMM LastMeasurements":dbl[](array[numeric])
  out "Graph DMMs 2":T4(graph) caption="XY Graph"
  out "DMMFileName":string
  out "error out (DMMs)":errorcluster={"status"=TRUE, "code"=-1074000000, "source"="ADCMT7351_ADC.lvlib:Error Query.vi<ERR>\nInstrument reports:\n+150,\"Illegal packet received\"\r\n+0,\"No error\"\r\n\n\n\n<b>Complete call chain:</b>\r\n     ADCMT7351_ADC.lvlib:Error Query.vi\r\n     DMMsData.lvclass:DDMs_low_measure.vi\r\n     DMMsData.lvclass:DMMs_measure.vi\r\n     CRYO_MASTER_FULL_dev.vi"}
  out "cycle # (DMMs)":i32
  in  "DMMsConfig":T13(array[cluster])=[{"Label"="I_H2", "Active?"=TRUE, "VISA resource name"="USB0::0x1334::0x0204::262800066::INSTR", "Device"=enum."ADCMT7351", "Measurement"=enum."DC Currents", "FileFormat"="%4.6e"}, {"Label"="V_H2", "Active?"=TRUE, "VISA resource name"="USB0::0x1334::0x0204::262800451::INSTR", "Device"=enum."ADCMT7351", "Measurement"=enum."DC Volts", "FileFormat"="%4.6e"}]
  in  "Measurement Interval DMMs (ms)":i64=500
  in  "InstName DMMs":string="DMMs"
  in  "Initialize (DMMs)":bool
  out "Graph DMMs 1":T4(graph) caption="XY Graph"
  out "error out (DMM graphs)":errorcluster
  in  "Sample #":i32=5
  in  "index T_ 1":i64=6
  in  "index T_2":i64=9
  out "error out (DMMs) 2":errorcluster={"status"=TRUE, "code"=-1074000000, "source"="ADCMT7351_ADC.lvlib:Error Query.vi<ERR>\nInstrument reports:\n+150,\"Illegal packet received\"\r\n+0,\"No error\"\r\n\n\n\n<b>Complete call chain:</b>\r\n     ADCMT7351_ADC.lvlib:Error Query.vi\r\n     DMMsData.lvclass:DDMs_low_measure.vi\r\n     DMMsData.lvclass:DMMs_measure.vi\r\n     CRYO_MASTER_FULL_dev.vi"}
  out "P_HEX7OUT":dbl=99725.65878507763 format="%_4e"
  out "P (HEX7 out)":dbl=99725.65878507763 format="%_4e"
  out "DP HEX5":dbl=144.28132689249568 format="%_4e"
  out "DP_HEX5":dbl=144.28132689249568 format="%_4e"
  in  "Diff pressure HEX5":string="DP_HEX5"
  out "3He pot level":dbl=0.2579228899986541 format="%_4f"
  in  "3He pot":string="L1"
  out "He level (3He)":dbl(slide)=0.2579228899986541 scale=0.0..100.0
  out "He level (1K) b":dbl(slide)=46.226026729665286 scale=0.0..100.0
  out "He level (1K)":dbl(slide)=49.88771505272982 scale=0.0..100.0
  out "He level (4K)":dbl(slide)=0.05537433565456876 scale=0.0..100.0
  out "1K pot(b1)":dbl=46.226026729665286 format="%_4f"
  in  "1K pot (b)":string="L2-2"
  in  "1K pot level":string="L2-1"
  out "L(1K) (a1)":dbl=49.88771505272982 format="%_4f"
  in  "SensorLocation 2":T14(ring)=enum."T3He5"
  out "Temperature 2":dbl=4.3215
  out "DP HEX4":dbl=-42.27649010016066 format="%_4e"
  in  "Diff pressure HEX4":string="DP_HEX4"
  out "V2":bool
  out "V1":bool=TRUE
  out "F5 (1K pump ex.)":dbl=37.619829557129414 format="%_4f"
  out "F4 (3He in to HEX7)":dbl=-7.249983269540847 format="%_3f"
  out "F3 (4He rtn flw via HEX7)":dbl=-0.052681534547558584 format="%_4f"
  out "F1 (3He pump exhaust) flow":dbl=3.609913543945148 format="%_4f"
  out "P (Dewar)":dbl=100437.10701708468 format="%_4e"